vi "UHR-Fleezers Control (host) - 12.4.vi"() -> ()   [LabVIEW 2012] (continued)
            n735 = property on="Trap 1 (ON/OFF)" class="Bool (strict)"("Val(Sgnl)"=w1046) -> ()  [unwired: 2 in, 2 out]
            n736 = Array To Cluster(array=w1053) -> (cluster=w1052:cluster{"[0]":dbl, "[1]":dbl, "[2]":dbl})
            n737 = call "Set Stage Position.vi"("Position"=w1052, "error in"=w1047, "VISA resource name in"=w1048) -> ("error out"=w1051:errorcluster)  [unwired: 2 out]
            n738 = local write "Stage Control Serial Error"(w1051) -> ()
          }
          frame #2 {
            n739 = local write "Stage Moving"(FALSE ("Stage Moving")) -> ()
            n740 = call <vilib>:"Beep.vi"() -> ()  [unwired: 3 in, 9 out]
            n741 = case shown="True" "Cap 2 Flow ON" {
              frame False {
              }
              frame True {
                n742 = property on="Inject Pump 3" class="Bool (strict)"("Val(Sgnl)"=TRUE ("Value (Signaling)")) -> ()  [unwired: 2 in, 2 out]
              }
            }
          }
          frame #3 {
            n743 = property on="Sample Channel\nFlow" class="Bool (strict)"("Val(Sgnl)"=FALSE ("Value (Signaling)")) -> ()  [unwired: 2 in, 2 out]
            n744 = case shown="False" "Cap. 2 BD T1?\n(ADig T1, DNA T2)" {
              tunnel: "Cap 2 T ON" -> [w1067 w1068]
              frame False {
                n745 = property on="Trap 2 (ON/OFF)" class="Bool (strict)"("Val(Sgnl)"=w1067) -> ()  [unwired: 2 in, 2 out]
              }
              frame True {
                n746 = property on="Trap 1 (ON/OFF)" class="Bool (strict)"("Val(Sgnl)"=w1068) -> ()  [unwired: 2 in, 2 out]
              }
            }
            n747 = property on="Got ADig bead" class="Bool"("Key Focus"=TRUE) -> ()  [unwired: 2 in, 2 out]
          }
        }
      }
      event "Initialize Blue Laser": Value Change {
        n748 = event-data() -> ()  [unwired: 1 in, 5 out]
        n749 = flat-sequence {
          tunnel: w1069 -> [w1088]
          frame #0 {
            n750 = Concatenate Strings("slmp ", "Modulation\nPower (mW)") -> (w1087:string)
            n751 = call "serial write macro.vi"("String"=w1087, "Delay (ms)"="Delay (ms)", "VISA resource name"=w1088) -> ("read buffer"=w1076:string, "error out"=w1077:errorcluster, "VISA resource name out"=w1084:refnum<visa-resource-name>)
            n752 = local write "read blue buffer"(w1076) -> ()
            n753 = local write "Blue Error Out"(w1077) -> ()
            n754 = call "serial write macro.vi"("String"="sdmes 1", "Delay (ms)"="Delay (ms)", "VISA resource name"=w1084) -> ("read buffer"=w1074:string, "error out"=w1075:errorcluster, "VISA resource name out"=w1082:refnum<visa-resource-name>)
            n755 = local write "Blue Error Out"(w1075) -> ()
            n756 = local write "read blue buffer"(w1074) -> ()
            n757 = call "serial write macro.vi"("String"="sames 1", "Delay (ms)"="Delay (ms)", "VISA resource name"=w1082) -> ("read buffer"=w1071:string, "error out"=w1073:errorcluster, "VISA resource name out"=w1079:refnum<visa-resource-name>)
            n758 = local write "read blue buffer"(w1071) -> ()
            n759 = local write "Blue Error Out"(w1073) -> ()
            n760 = call "serial write macro.vi"("String"="l1", "Delay (ms)"="Delay (ms)", "VISA resource name"=w1079) -> ("read buffer"=w1070:string, "error out"=w1072:errorcluster)  [unwired: 1 out]
            n761 = local write "read blue buffer"(w1070) -> ()
            n762 = local write "Blue Error Out"(w1072) -> ()
          }
          frame #1 {
            n763 = local write "Initialize Blue Laser"(FALSE ("Initialize")) -> ()
          }
        }
      }
      event "Send string\nto Blue Laser": Value Change {
        n764 = event-data() -> ()  [unwired: 1 in, 5 out]
        n765 = flat-sequence {
          tunnel: w1090 -> [w1095]
          frame #0 {
            n766 = local read "Delay (ms)"() -> (w1092:i32)
            n767 = call "serial write macro.vi"("String"="command string", "Delay (ms)"=w1092, "VISA resource name"=w1095) -> ("read buffer"=w1093:string, "error out"=→"Blue Error Out":errorcluster)  [unwired: 1 out]
            "read blue buffer" <- w1093
            n768 = String Length(string=w1093) -> (length=→"length":i32)
            "command string sent" <- "command string"
          }
          frame #1 {
            n769 = local write "Send string\nto Blue Laser"(FALSE ("Send string")) -> ()
          }
        }
      }
      event "Read Harvard": Value Change {
        n770 = event-data() -> ()  [unwired: 1 in, 5 out]
        n771 = Concatenate Strings("write buffer", "\r") -> (w1102:string)
        n772 = VISA Write(VISA resource name=w1100, write buffer=w1102, error in (no error)=w1099) -> (VISA resource name out=w1111:refnum<visa-resource-name>, error out=w1110:errorcluster)  [unwired: 1 out]
        n773 = stacked-sequence {
          tunnel: [w1114] -> w1109
          tunnel: w1111 -> [w1114]
          tunnel: w1110 -> [w1113]
          tunnel: [w1113] -> w1104
          frame #0 {
            n774 = Wait (ms)(milliseconds to wait=50) -> ()  [unwired: 1 out]
          }
        }
        n775 = property class="Instr"(reference=w1109, error in=w1104) -> (reference out=w1108:refnum<visa-resource-name>, error out=w1106:errorcluster, "Serial Settings:Number of Bytes at Serial Port"=w1107:u32)
        "Serial Settings:Number of Bytes at Serial Port" <- w1107
        n776 = VISA Read(VISA resource name=w1108, byte count=w1107, error in (no error)=w1106) -> (read buffer=w1105:string)  [unwired: 3 out]
        "read buffer" <- w1105
        n777 = Fract/Exp String To Number(string=w1105) -> ()  [unwired: 5 out]
      }
      event "+z", "-z": Value Change {
        n778 = event-data() -> ()  [unwired: 1 in, 5 out]
        n779 = flat-sequence {
          tunnel: w1115 -> [w1137]
          tunnel: w1116 -> [w1117]
          frame #0 {
            n780 = call "Read Stage Position.vi"("error in"=w1137, "VISA resource name in"=w1117) -> ("Current Position"=w1122:cluster{dbl, dbl, dbl}, "error out"=w1135:errorcluster, "VISA resource name out"=w1136:refnum<visa-resource-name>)  [unwired: 1 out]
            n781 = local read "Saved Stage Positions"() -> (w1146:dbl[][])
            n782 = Divide(x="z nudge increment (um)", y=1000.0) -> (x/y=w1134:dbl)
            n783 = Boolean To (0,1)(Boolean="+z") -> (0, 1=w1126:i16)
            n784 = Boolean To (0,1)(Boolean="-z") -> (0, 1=w1127:i16)
            n785 = Array Subset(array=w1146, index (row)=1 ("index"), length (row)=1 ("length"), index (col)=1 ("index"), length (col)=3 ("length")) -> (w1143:dbl[][])
            n786 = Multiply(x=w1126, y=w1134) -> (x*y=w1130:dbl)
            n787 = Multiply(x=w1127, y=w1134) -> (x*y=w1128:dbl)
            n788 = Unbundle(w1122) -> (w1120:dbl, w1119:dbl, w1123:dbl)
            n789 = Negate(x=w1128) -> (-x=w1129:dbl)
            n790 = Reshape Array(w1143, 3 ("dimension size")) -> (w1141:dbl[])
            n791 = Add(x=w1130, y=w1129) -> (x+y=w1131:dbl)
            n792 = Array To Cluster(array=w1141) -> ()  [unwired: 1 out]
            n793 = Add(x=w1131, y=w1123) -> (x+y=w1121:dbl)
            n794 = Bundle(cluster=w1122, w1120, w1119, w1121) -> (w1118:cluster{dbl, dbl, dbl})
            n795 = call "Set Stage Position.vi"("Position"=w1118, "error in"=w1135, "VISA resource name in"=w1136) -> ("error out"=w1140:errorcluster)  [unwired: 2 out]
            n796 = local write "Stage Moving"(TRUE ("Stage Moving")) -> ()
            n797 = local write "Stage Control Serial Error"(w1140) -> ()
          }
          frame #1 {
            n798 = local write "Stage Moving"(FALSE ("Stage Moving")) -> ()
            n799 = call <vilib>:"Beep.vi"() -> ()  [unwired: 3 in, 9 out]
          }
        }
      }
      event "Cal/Data Acq. Spot": Value Change {
        n800 = event-data() -> ()  [unwired: 1 in, 5 out]
        n801 = flat-sequence {
          tunnel: w1155 -> [w1159]
          tunnel: w1156 -> [w1160]
          tunnel: [w1160] -> w1152
          tunnel: [w1159] -> w1151
          tunnel: w1152 -> [w1165]
          tunnel: w1151 -> [w1164]
          tunnel: ["Cal @ (MHz)"] -> w1149
          tunnel: [w1169] -> w1153
          tunnel: w1149 -> [w1169]
          tunnel: w1153 -> [w1178]
          tunnel: ["W/ Offset 1"] -> w1150
          tunnel: w1153 -> [w1199]
          tunnel: w1150 -> [w1197]
          frame #0 {
            n802 = property on="Sample Channel\nFlow" class="Bool (strict)"("Val(Sgnl)"="Daq spot flow on") -> ()  [unwired: 2 in, 2 out]
            n803 = Wait (ms)(milliseconds to wait=u32 250) -> ()  [unwired: 1 out]
          }
          frame #1 {
            n804 = local read "Saved Stage Positions"() -> (w1162:dbl[][])
            n805 = property on="Trap Delta (MHz)" class="DigNum (strict)"("Val(Sgnl)"="Cal @ (MHz)") -> ()  [unwired: 2 in, 2 out]
            n806 = local write "Stage Moving"(TRUE ("Stage Moving")) -> ()
            n807 = call "move to saved stage position.vi"("error in"=w1164, "Stage VISA resource name in"=w1165, "Position"="Cal Stage Position", "Saved Stage Positions"=w1162) -> ("error out"=w1163:errorcluster)  [unwired: 1 out]
            n808 = local write "Stage Control Serial Error"(w1163) -> ()
          }
          frame #2 {
            n809 = local write "Stage Moving"(FALSE ("Stage Moving")) -> ()
            n810 = property on="Sample Channel\nFlow" class="Bool (strict)"("Val(Sgnl)"="Flow ON during cal?") -> ()  [unwired: 2 in, 2 out]
            n811 = call <vilib>:"Beep.vi"() -> ()  [unwired: 3 in, 9 out]
          }
          frame #3 {
            n812 = Wait (ms)(milliseconds to wait=u32 1000) -> ()  [unwired: 1 out]
          }
          frame #4 {
            n813 = property on="Save Calibration" class="Bool (strict)"("Val(Sgnl)"=TRUE ("Value (Signaling)")) -> ()  [unwired: 2 in, 2 out]
          }
          frame #5 {
            n814 = Wait (ms)(milliseconds to wait=u32 2000) -> ()  [unwired: 1 out]
          }
          frame #6 {
            # "Check to see if \nsaving done"
            n815 = while {
              stop <- w1174 stop-if-true
              n816 = local read "Saving..."() -> (w1175:bool)
              n817 = Wait (ms)(milliseconds to wait=u32 100) -> ()  [unwired: 1 out]
              n818 = Not(x=w1175) -> (.not. x?=w1174:bool)
            }
          }
          frame #7 {
            n819 = case shown="True" "W/ Offset 1" {
              tunnel: w1178 -> [_ w1179]
              frame False {
              }
              frame True {
                n820 = stacked-sequence {
                  tunnel: w1179 -> [_ _ _ _ _ _ _ w1196]
                  frame #0 {
                    n821 = property on="Trap Delta (MHz)" class="DigNum (strict)"("Val(Sgnl)"="Offset 1 Start (MHz)") -> ()  [unwired: 2 in, 2 out]
                    n822 = Replace Array Subset(array=u32[] [0] ("Index Values"), new element="Offset 1 Set", index=0) -> (w1180:u32[])
                    n823 = property on="Saved AOD Raster Scan Parameter Sets" class="Arr (strict)"("Index Values"=w1180) -> ()  [unwired: 2 in, 2 out]
                  }
                  frame #1 {
                    n824 = Wait (ms)(milliseconds to wait=u32 200) -> ()  [unwired: 1 out]
                  }
                  frame #2 {
                    n825 = property on="Load parameters" class="Bool (strict)"("Val(Sgnl)"=TRUE ("Value (Signaling)")) -> ()  [unwired: 2 in, 2 out]
                  }
                  frame #3 {
                    n826 = Wait (ms)(milliseconds to wait=u32 200) -> ()  [unwired: 1 out]
                  }
                  frame #4 {
                    n827 = property on="Trap Raster Scan" class="Bool (strict)"("Val(Sgnl)"=TRUE ("Value (Signaling)")) -> ()  [unwired: 2 in, 2 out]
                  }
                  frame #5 {
                    n828 = Wait (ms)(milliseconds to wait=u32 2000) -> ()  [unwired: 1 out]
                  }
                  frame #6 {
                    n829 = while {
                      stop <- w1193 stop-if-true
                      n830 = local read "Raster Scanning..."() -> (w1195:bool)
                      n831 = local read "Saving..."() -> (w1191:bool)
                      n832 = Wait (ms)(milliseconds to wait=u32 100) -> ()  [unwired: 1 out]
                      n833 = Not(x=w1191) -> (.not. x?=w1190:bool)
                      n834 = Not(x=w1195) -> (.not. x?=w1192:bool)
                      n835 = And(x=w1192, y=w1190) -> (x .and. y?=w1193:bool)
                    }
                  }
                  frame #7 {
                    n836 = property on="Trap Delta (MHz)" class="DigNum (strict)"("Val(Sgnl)"=w1196) -> ()  [unwired: 2 in, 2 out]
                  }
                }
              }
            }
          }
          frame #8 {
            n837 = local read "Save ave N"() -> (w1198:dbl)
            n838 = case shown="False" "W/ Offset 2" {
              tunnel: w1199 -> [_ w1206]
              tunnel: w1198 -> [_ w1205]
              tunnel: w1197 -> [w1201 _]
              frame False {
                n839 = case shown="False" w1201 {
                  frame False {
                    n840 = Multiply(x="Cal read wait (s)", y=u32 1000 ("milliseconds to wait")) -> (x*y=w1203:u32)
                    n841 = Wait (ms)(milliseconds to wait=w1203) -> ()  [unwired: 1 out]
                  }
                  frame True {
                  }
                }
              }
              frame True {
                n842 = stacked-sequence {
                  tunnel: w1206 -> [_ _ _ _ _ _ _ _ _ w1227 _ _]
                  tunnel: w1205 -> [_ _ _ _ _ _ _ _ _ w1225 _ _]
                  frame #0 {
                    n843 = property on="Save ave N" class="DigNum (strict)"("Val(Sgnl)"=1.0 ("Value (Signaling)")) -> ()  [unwired: 2 in, 2 out]
                  }
                  frame #1 {
                    n844 = Wait (ms)(milliseconds to wait=u32 500) -> ()  [unwired: 1 out]
                  }
                  frame #2 {
                    n845 = property on="Trap Delta (MHz)" class="DigNum (strict)"("Val(Sgnl)"="Offset 2 Start (MHz)") -> ()  [unwired: 2 in, 2 out]
                    n846 = Replace Array Subset(array=u32[] [0] ("Index Values"), new element="Offset 2 Set", index=0) -> (w1211:u32[])
                    n847 = property on="Saved AOD Raster Scan Parameter Sets" class="Arr (strict)"("Index Values"=w1211) -> ()  [unwired: 2 in, 2 out]
                  }
                  frame #3 {
                    n848 = Wait (ms)(milliseconds to wait=u32 500) -> ()  [unwired: 1 out]
                  }
                  frame #4 {
                    n849 = property on="Load parameters" class="Bool (strict)"("Val(Sgnl)"=TRUE ("Value (Signaling)")) -> ()  [unwired: 2 in, 2 out]
                  }
                  frame #5 {
                    n850 = Wait (ms)(milliseconds to wait=u32 500) -> ()  [unwired: 1 out]
                  }
                  frame #6 {
                    n851 = property on="Trap Raster Scan" class="Bool (strict)"("Val(Sgnl)"=TRUE ("Value (Signaling)")) -> ()  [unwired: 2 in, 2 out]
                  }
                  frame #7 {
                    n852 = Wait (ms)(milliseconds to wait=u32 2000) -> ()  [unwired: 1 out]
                  }
                  frame #8 {
                    n853 = while {
                      stop <- w1220 stop-if-true
                      n854 = local read "Raster Scanning..."() -> (w1223:bool)
                      n855 = local read "Saving..."() -> (w1221:bool)
                      n856 = Wait (ms)(milliseconds to wait=u32 100) -> ()  [unwired: 1 out]
                      n857 = Not(x=w1221) -> (.not. x?=w1219:bool)
                      n858 = Not(x=w1223) -> (.not. x?=w1222:bool)
                      n859 = And(x=w1222, y=w1219) -> (x .and. y?=w1220:bool)
                    }
                  }
                  frame #9 {
                    n860 = property on="Trap Delta (MHz)" class="DigNum (strict)"("Val(Sgnl)"=w1227) -> ()  [unwired: 2 in, 2 out]
                    n861 = property on="Saved AOD Raster Scan Parameter Sets" class="Arr (strict)"("Index Values"=u32[] [0]) -> ()  [unwired: 2 in, 2 out]
                    n862 = property on="Save ave N" class="DigNum (strict)"("Val(Sgnl)"=w1225) -> ()  [unwired: 2 in, 2 out]
                  }
                  frame #10 {
                    n863 = Wait (ms)(milliseconds to wait=u32 500) -> ()  [unwired: 1 out]
                  }
                  frame #11 {
                    n864 = property on="Load parameters" class="Bool (strict)"("Val(Sgnl)"=TRUE ("Value (Signaling)")) -> ()  [unwired: 2 in, 2 out]
                  }
                }
              }
            }
          }
          frame #9 {
            n865 = property on="Read Cal" class="Bool (strict)"("Val(Sgnl)"=TRUE ("Value (Signaling)")) -> ()  [unwired: 2 in, 2 out]
          }
          frame #10 {
            n866 = Wait (ms)(milliseconds to wait=u32 1000) -> ()  [unwired: 1 out]
          }
          frame #11 {
            n867 = property on="Fish for Tether" class="Bool (strict)"("Val(Sgnl)"=TRUE ("Value (Signaling)")) -> ()  [unwired: 2 in, 2 out]
          }
        }
        n868 = local write "Cal/Data Acq. Spot"(FALSE ("Cal/Data Acq. Spot")) -> ()
      }
      event "Dump Beads": Value Change {
        n869 = event-data() -> ()  [unwired: 1 in, 5 out]
        n870 = flat-sequence {
          tunnel: ["Dump spot flow on?"] -> w1233
          tunnel: [w1244] -> w1234
          tunnel: w1233 -> [w1244]
          tunnel: w1237 -> [w1249]
          tunnel: w1236 -> [w1248]
          tunnel: [w1246] -> w1235
          tunnel: w1234 -> [w1246]
          tunnel: w1235 -> [w1259]
          frame #0 {
            w1238 = FALSE ("Value (Signaling)")
            n871 = local read "Saving..."() -> (w1240:bool)
            n872 = local write "Dump Beads"(FALSE ("Dump Beads")) -> ()
            n873 = property on="Inject Pump 3" class="Bool (strict)"("Val(Sgnl)"=w1238) -> ()  [unwired: 2 in, 2 out]
            n874 = property on="Inject Pump 1" class="Bool (strict)"("Val(Sgnl)"=w1238) -> ()  [unwired: 2 in, 2 out]
            n875 = local write "Stop Saving"(w1240) -> ()
          }
          frame #1 {
            w1241 = FALSE ("Fl. Triggered...")
            n876 = case shown="True" "Dump spot flow on?" {
              frame False {
              }
              frame True {
                n877 = property on="Sample Channel\nFlow" class="Bool (strict)"("Val(Sgnl)"=TRUE ("Stage Moving")) -> ()  [unwired: 2 in, 2 out]
              }
            }
            n878 = local write "Fl. Triggered..."(w1241) -> ()
            n879 = local write "Tether"(w1241) -> ()
            n880 = property on="Green Laser ON" class="Bool (strict)"("Val(Sgnl)"=w1241) -> ()  [unwired: 2 in, 2 out]
            n881 = property on="Trap Pos. FB ON" class="Bool (strict)"("Val(Sgnl)"=w1241) -> ()  [unwired: 2 in, 2 out]
            n882 = property on="Trap Trig. Fl." class="Bool (strict)"("Val(Sgnl)"=w1241) -> ()  [unwired: 2 in, 2 out]
            n883 = property on="Fl. Triggered..." class="Bool (strict)"("Val(Sgnl)"=w1241) -> ()  [unwired: 2 in, 2 out]
            n884 = property on="Dip for Protein" class="Bool (strict)"("Val(Sgnl)"=w1241) -> ()  [unwired: 2 in, 2 out]
            n885 = property on="Pause dwell" class="Bool (strict)"("Val(Sgnl)"=w1241) -> ()  [unwired: 2 in, 2 out]
          }
          frame #2 {
            n886 = property on="Trap Pos. FB Offset Factor" class="DigNum (strict)"("Val(Sgnl)"=i64 0 ("Value (Signaling)")) -> ()  [unwired: 2 in, 2 out]
          }
          frame #3 {
            n887 = local read "Saved Stage Positions"() -> (w1250:dbl[][])
            n888 = local write "Stage Moving"(TRUE ("Stage Moving")) -> ()
            n889 = Array Subset(array=w1250, index (row)=3 ("index"), length (row)=1 ("length"), index (col)=1 ("index"), length (col)=3 ("length")) -> (w1255:dbl[][])
            n890 = Reshape Array(w1255, 3 ("dimension size")) -> (w1253:dbl[])
            n891 = Array To Cluster(array=w1253) -> (cluster=w1252:cluster{"[0]":dbl, "[1]":dbl, "[2]":dbl})
            n892 = call "Set Stage Position.vi"("Position"=w1252, "error in"=w1248, "VISA resource name in"=w1249) -> ()  [unwired: 3 out]
          }
          frame #4 {
            w1260 = FALSE ("Value (Signaling)")
            n893 = case shown="True" w1259 {
              frame False {
              }
              frame True {
                n894 = property on="Sample Channel\nFlow" class="Bool (strict)"("Val(Sgnl)"=FALSE ("Stage Moving")) -> ()  [unwired: 2 in, 2 out]
              }
            }
            n895 = property on="Trap 1 (ON/OFF)" class="Bool (strict)"("Val(Sgnl)"=w1260) -> ()  [unwired: 2 in, 2 out]
            n896 = property on="Trap 2 (ON/OFF)" class="Bool (strict)"("Val(Sgnl)"=w1260) -> ()  [unwired: 2 in, 2 out]
            n897 = call <vilib>:"Beep.vi"() -> ()  [unwired: 3 in, 9 out]
          }
          frame #5 {
            n898 = property on="Move Cap. 2 (ADig Top)" class="Bool (strict)"("Val(Sgnl)"=TRUE ("Value (Signaling)")) -> ()  [unwired: 2 in, 2 out]
            n899 = property on="Tab Control" class="TabCtl (strict)"("Val(Sgnl)"=T25."Status" ("Value (Signaling)")) -> ()  [unwired: 2 in, 2 out]
          }
        }
      }
      event "Dip for Protein": Value Change {
        n900 = event-data() -> ()  [unwired: 1 in, 5 out]
        n901 = case shown="True" "Dip for Protein" {
          tunnel: w1266 -> [_ w1268]
          tunnel: w1265 -> [_ w1267]
          frame False {
          }
          frame True {
            n902 = while {
              tunnel: w1268 -> [w1279]
              tunnel: w1267 -> [w1278]
              i -> [w1273]
              stop <- w1275 stop-if-true
              n903 = Increment(x=w1273) -> (x+1=→"Dip #":i32)
              n904 = flat-sequence {
                tunnel: w1278 -> [w1290]
                tunnel: w1279 -> [w1291]
                tunnel: [w1291] -> w1283
                tunnel: [w1290] -> w1282
                tunnel: [w1284] -> w1269
                tunnel: [w1296] -> w1277
                tunnel: [w1297] -> w1276
                tunnel: w1283 -> [w1298]
                tunnel: w1282 -> [w1299]
                tunnel: [w1294] -> w1270
                tunnel: w1269 -> [w1294]
                tunnel: [w1307] -> w1281
                tunnel: w1277 -> [w1307]
                tunnel: [w1306] -> w1280
                tunnel: w1276 -> [w1306]
                tunnel: [w1303] -> w1274
                tunnel: [w1302] -> w1271
                tunnel: w1270 -> [w1302]
                tunnel: w1280 -> [w1327]
                tunnel: w1281 -> [w1328]
                tunnel: w1274 -> [w1329]
                tunnel: w1271 -> [w1326]
                tunnel: [w1385] -> w1275
                frame #0 {
                  n905 = local read "Trap Pos. FB ON"() -> (w1284:bool)
                  n906 = Compound Arithmetic op=AND("Flow ON\nduring dip?", "FB OFF when \nflow ON", w1284) -> (w1285:bool)
                  n907 = case shown="True" "Move trap \nbefore dip move?" {
                    frame False {
                    }
                    frame True {
                      n908 = property on="Trap Delta (MHz)" class="DigNum (strict)"("Val(Sgnl)"="Dipping Delta (MHz)") -> ()  [unwired: 2 in, 2 out]
                    }
                  }
                  n909 = property on="Green Laser ON" class="Bool (strict)"("Val(Sgnl)"="Green ON\nbefore dip?") -> ()  [unwired: 2 in, 2 out]
                  n910 = property on="Sample Channel\nFlow" class="Bool (strict)"("Val(Sgnl)"="Flow ON\nduring dip?") -> ()  [unwired: 2 in, 2 out]
                  n911 = case shown="True" w1285 {
                    frame False {
                    }
                    frame True {
                      n912 = property on="Trap Pos. FB ON" class="Bool (strict)"("Val(Sgnl)"=FALSE ("Value (Signaling)")) -> ()  [unwired: 2 in, 2 out]
                    }
                  }
                }
                frame #1 {
                  n913 = local read "Saved Stage Positions"() -> (w1301:dbl[][])
                  n914 = local write "Cancel dwell"(FALSE ("Cancel dwell")) -> ()
                  n915 = call "move to saved stage position.vi"("error in"=w1299, "Stage VISA resource name in"=w1298, "Position"="Dip Stage \nPosition", "Saved Stage Positions"=w1301) -> ("VISA resource name out"=w1296:refnum<visa-resource-name>, "error out"=w1297:errorcluster)
                }
                frame #2 {
                  n916 = node-c288() -> (w1305:T22)  [unwired: 4 in]
                  n917 = timed-loop {
                    timing: w1305 -> [_]
                    timing-out: [_] -> w1304
                    tunnel: [w1311] -> w1303
                    i -> [w1308]
                    stop <- w1312 stop-if-true
                    n918 = node-c288() -> ()  [unwired: 1 in, 1 out]
                    n919 = Greater Or Equal?(x=w1308, y="Dip Duration (s)") -> (x >= y?=w1320:bool)
                    n920 = local read "Dip for Protein"() -> (w1313:bool)
                    n921 = local read "Dump Beads"() -> (w1310:bool)
                    n922 = local read "Cancel dwell"() -> (w1319:bool)
                    n923 = local read "Pause dwell"() -> (w1316:bool)
                    n924 = Not(x=w1313) -> (.not. x?=w1318:bool)
                    n925 = Compound Arithmetic op=OR(w1319, w1320, w1318) -> (w1317:bool)
                    n926 = Select(t=FALSE, s=w1316, f=w1317) -> (s? t:f=w1314:bool)
                    n927 = Not(x=w1310) -> (.not. x?=w1309:bool)
                    n928 = node-c288() -> ()  [unwired: 1 in, 1 out]
                    n929 = And(x=w1313, y=w1309) -> (x .and. y?=w1311:bool)
                    n930 = Or(x=w1314, y=w1310) -> (x .or. y?=w1312:bool)
                    "Dip Time (s)" <- w1308
                  }
                  n931 = node-c288(w1304) -> ()  [unwired: 1 out]
                }
                frame #3 {
                  n932 = case shown="True" w1329 {
                    tunnel: w1328 -> [_ w1334]
                    tunnel: w1327 -> [_ w1333]
                    tunnel: w1326 -> [_ w1330]
                    frame False {
                    }
                    frame True {
                      n933 = flat-sequence {
                        tunnel: w1333 -> [w1338]
                        tunnel: w1334 -> [w1339]
                        tunnel: [w1339] -> w1332
                        tunnel: [w1338] -> w1331
                        tunnel: w1330 -> [w1335]
                        tunnel: w1332 -> [w1349]
                        tunnel: w1331 -> [w1348]
                        tunnel: w1330 -> [w1357]
                        frame #0 {
                          n934 = local read "Sample Channel\nFlow"() -> (w1337:bool)
                          n935 = case shown="True" w1337 {
                            tunnel: "Flow ON \nduring return\nfrom dip?" -> [w1340 w1343]
                            tunnel: w1335 -> [_ w1342]
                            frame False {
                              n936 = case shown="True" w1340 {
                                frame False {
                                }
                                frame True {
                                n937 = property on="Sample Channel\nFlow" class="Bool (strict)"("Val(Sgnl)"=TRUE ("Value (Signaling)")) -> ()  [unwired: 2 in, 2 out]
                                }
                              }
                            }
                            frame True {
                              n938 = case shown="False" w1343 {
                                tunnel: w1342 -> [w1344 _]
                                frame False {
                                n939 = property on="Trap Pos. FB ON" class="Bool (strict)"("Val(Sgnl)"=w1344) -> ()  [unwired: 2 in, 2 out]
                                n940 = property on="Sample Channel\nFlow" class="Bool (strict)"("Val(Sgnl)"=FALSE ("Value (Signaling)")) -> ()  [unwired: 2 in, 2 out]
                                }
                                frame True {
                                }
                              }
                            }
                          }
                        }
                        frame #1 {
                          # "For turning on green laser before stage reaches lower spot"
                          n941 = case shown="True" "Green ON\nafter start\nreturn?" {
                            frame False {
                            }
                            frame True {
                              n942 = flat-sequence {
                                frame #0 {
                                n943 = Multiply(x="Green delay after \nstart return (s)", y=1000.0) -> (x*y=w1354:dbl)
                                n944 = Wait (ms)(milliseconds to wait=w1354) -> ()  [unwired: 1 out]
                                }
                                frame #1 {
                                n945 = property on="Green Laser ON" class="Bool (strict)"("Val(Sgnl)"=TRUE ("Value (Signaling)")) -> ()  [unwired: 2 in, 2 out]
                                }
                              }
                            }
                          }
                          n946 = local read "Saved Stage Positions"() -> (w1352:dbl[][])
                          n947 = local write "Cancel dwell"(FALSE ("Cancel dwell")) -> ()
                          n948 = call "move to saved stage position.vi"("error in"=w1348, "Stage VISA resource name in"=w1349, "Position"="Return Stage \nPosition", "Saved Stage Positions"=w1352) -> ("error out"=w1350:errorcluster)  [unwired: 1 out]
                          n949 = local write "Stage Control Serial Error"(w1350) -> ()
                        }
                        frame #2 {
                          n950 = property on="Trap Pos. FB ON" class="Bool (strict)"("Val(Sgnl)"=w1357) -> ()  [unwired: 2 in, 2 out]
                          n951 = case shown="True" "Green ON \nafter return?" {
                            frame False {
                            }
                            frame True {
                              n952 = property on="Green Laser ON" class="Bool (strict)"("Val(Sgnl)"=TRUE ("Value (Signaling)")) -> ()  [unwired: 2 in, 2 out]
                            }
                          }
                          n953 = case shown="True" "Move trap after return?" {
                            frame False {
                            }
                            frame True {
                              n954 = property on="Trap Delta (MHz)" class="DigNum (strict)"("Val(Sgnl)"="Dip Trap Delta 2 (MHz)") -> ()  [unwired: 2 in, 2 out]
                            }
                          }
                          n955 = case shown="True" "Save data after return?" {
                            frame False {
                            }
                            frame True {
                              n956 = property on="Start Saving" class="Bool (strict)"("Val(Sgnl)"=TRUE ("Value (Signaling)")) -> ()  [unwired: 2 in, 2 out]
                            }
                          }
                          n957 = property on="Sample Channel\nFlow" class="Bool (strict)"("Val(Sgnl)"="Flow ON\nduring daq?") -> ()  [unwired: 2 in, 2 out]
                        }
                        frame #3 {
                          n958 = node-c288() -> (w1366:T22)  [unwired: 4 in]
                          n959 = timed-loop {
                            timing: w1366 -> [_]
                            timing-out: [_] -> w1365
                            i -> [w1367]
                            stop <- w1369 stop-if-true
                            n960 = node-c288() -> ()  [unwired: 1 in, 1 out]
                            n961 = local read "Dump Beads"() -> (w1368:bool)
                            n962 = Greater Or Equal?(x=w1367, y="Dwell Duration (s)") -> (x >= y?=w1374:bool)
                            n963 = local read "Dip for Protein"() -> (w1371:bool)
                            n964 = Not(x=w1371) -> (.not. x?=w1370:bool)
                            n965 = Compound Arithmetic op=OR(w1374, "Cancel dwell", w1370) -> (w1373:bool)
                            n966 = node-c288() -> ()  [unwired: 1 in, 1 out]
                            n967 = Select(t=FALSE, s="Pause dwell", f=w1373) -> (s? t:f=w1376:bool)
                            n968 = Or(x=w1376, y=w1368) -> (x .or. y?=w1369:bool)
                            "Dwell Time (s)" <- w1367
                          }
                          n969 = node-c288(w1365) -> ()  [unwired: 1 out]
                        }
                      }
                    }
                  }
                }
                frame #4 {
                  n970 = local read "Dip for Protein"() -> (w1386:bool)
                  n971 = local read "Dump Beads"() -> (w1383:bool)
                  n972 = local write "Cancel dwell"(FALSE ("Cancel dwell")) -> ()
                  n973 = Not(x=w1386) -> (.not. x?=w1387:bool)
                  n974 = Not(x="Cont. Repeat Dipping?") -> (.not. x?=w1389:bool)
                  n975 = Compound Arithmetic op=OR(w1387, w1389, w1383) -> (w1385:bool)
                }
              }
            }
          }
        }
      }
      event "Profile": Value Change {
        n976 = event-data() -> ()  [unwired: 1 in, 5 out]
        n977 = flat-sequence {
          tunnel: w1398 -> [w1401]
          tunnel: w1397 -> [w1409]
          tunnel: [w1403] -> w1396
          tunnel: [w1402] -> w1395
          tunnel: [w1400] -> w1393
          tunnel: [w1399] -> w1390
          tunnel: w1396 -> [w1416]
          tunnel: w1395 -> [w1415]
          tunnel: [w1413] -> w1394
          tunnel: w1393 -> [w1414]
          tunnel: [w1412] -> w1392
          tunnel: [w1411] -> w1391
          tunnel: w1390 -> [w1411]
          tunnel: w1394 -> [w1420]
          tunnel: w1392 -> [w1419]
          tunnel: w1391 -> [w1418]
          frame #0 {
            n978 = call "Read Stage Position.vi"("error in"=w1409, "VISA resource name in"=w1401) -> ("Current Position"=w1399:cluster{dbl, dbl, dbl}, "error out"=w1402:errorcluster, "VISA resource name out"=w1400:refnum<visa-resource-name>)  [unwired: 1 out]
            "Current Position" <- w1399
            n979 = local write "Stage Control Serial Error"(w1402) -> ()
            n980 = Unbundle(w1399) -> (w1406:dbl, w1408:dbl, w1404:dbl)
            n981 = Add(x=w1408, y="Y change (mm)") -> (x+y=w1405:dbl)
            n982 = Bundle(w1406, w1405, w1404) -> (w1403:cluster{dbl, dbl, dbl})  [unwired: 1 in]
          }
          frame #1 {
            # "move to new position and start saving"
            n983 = local write "Stage Moving"(TRUE ("Stage Moving")) -> ()
            n984 = local write "Start Saving"(TRUE ("Start Saving")) -> ()
            n985 = call "Set Stage Position.vi"("Position"=w1416, "error in"=w1415, "VISA resource name in"=w1414) -> ("error out"=w1412:errorcluster, "VISA resource name out"=w1413:refnum<visa-resource-name>)  [unwired: 1 out]
          }
          frame #2 {
            # "go back to start"
            n986 = call "Set Stage Position.vi"("Position"=w1418, "error in"=w1419, "VISA resource name in"=w1420) -> ()  [unwired: 3 out]
          }
          frame #3 {
            # "stop saving"
            n987 = local write "Stop Saving"(TRUE ("Stop Saving")) -> ()
            n988 = local write "Stage Moving"(FALSE ("Stage Moving")) -> ()
          }
        }
      }
      event "Move to Position 1", "Move to Position 2", "Move to Position 3", "Move to Position 4", "Move to Position 5", "Lower Ch. Cap.": Value Change {
        n989 = event-data() -> ()  [unwired: 1 in, 5 out]
        n990 = Or(x="Move to Position 5", y="Lower Ch. Cap.") -> (x .or. y?=w1426:bool)
        n991 = Build Array("Move to Position 1", "Move to Position 2", "Move to Position 3", "Move to Position 4", w1426) -> (w1429:bool[])
        n992 = Boolean Array To Number(Boolean array=w1429) -> (number=w1428:u32)
        n993 = Logarithm Base 2(1:w1428) -> (0:w1427:dbl)
        n994 = flat-sequence {
          tunnel: w1427 -> [w1438]
          tunnel: w1424 -> [w1436]
          tunnel: w1423 -> [w1435]
          frame #0 {
            n995 = local read "Saved Stage Positions"() -> (w1446:dbl[][])
            n996 = Array Subset(array=w1446, index (row)=w1438, length (row)=1 ("length"), index (col)=1 ("index"), length (col)=3 ("length")) -> (w1443:dbl[][])
            n997 = Reshape Array(w1443, 3 ("dimension size")) -> (w1441:dbl[])
            n998 = Array To Cluster(array=w1441) -> (cluster=w1440:cluster{"[0]":dbl, "[1]":dbl, "[2]":dbl})
            n999 = call "Set Stage Position.vi"("Position"=w1440, "error in"=w1435, "VISA resource name in"=w1436) -> ("error out"=w1439:errorcluster)  [unwired: 2 out]
            n1000 = local write "Stage Moving"(TRUE ("Stage Moving")) -> ()
            n1001 = local write "Stage Control Serial Error"(w1439) -> ()
          }
          frame #1 {
            n1002 = local write "Stage Moving"(FALSE ("Stage Moving")) -> ()
            n1003 = call <vilib>:"Beep.vi"() -> ()  [unwired: 3 in, 9 out]
          }
        }
      }
      event "Got ADig bead": Value Change {
        n1004 = event-data() -> ()  [unwired: 1 in, 5 out]
        n1005 = flat-sequence {
          frame #0 {
            n1006 = local read "Cap 1 Samp Flow ON"() -> (w1450:bool)
            n1007 = case shown="True" w1450 {
              frame False {
              }
              frame True {
                n1008 = property on="Sample Channel\nFlow" class="Bool (strict)"("Val(Sgnl)"=TRUE ("Value (Signaling)")) -> ()  [unwired: 2 in, 2 out]
              }
            }
          }
          frame #1 {
            n1009 = property on="Inject Pump 3" class="Bool (strict)"("Val(Sgnl)"=FALSE ("Value (Signaling)")) -> ()  [unwired: 2 in, 2 out]
          }
          frame #2 {
            n1010 = property on="Move Cap. 1 (DNA Bottom)" class="Bool (strict)"("Val(Sgnl)"=TRUE ("Value (Signaling)")) -> ()  [unwired: 2 in, 2 out]
          }
        }
      }
      event "Force FB Data\nScript": Value Change {
        n1011 = event-data() -> ()  [unwired: 1 in, 5 out]
        n1012 = flat-sequence {
          tunnel: w1459 -> [w1463]
          tunnel: w1460 -> [w1464]
          tunnel: [w1464] -> w1455
          tunnel: [w1463] -> w1454
          tunnel: w1455 -> [w1467]
          tunnel: w1454 -> [w1466]
          tunnel: ["Trap Trig Fl."] -> w1456
          tunnel: [w1492] -> w1457
          tunnel: w1456 -> [w1492]
          tunnel: [w1496] -> w1458
          tunnel: w1457 -> [w1496]
          tunnel: w1458 -> [w1498]
          frame #0 {
            n1013 = property on="Trap Delta (MHz)" class="DigNum (strict)"("Val(Sgnl)"="Trap Delta Before Moving") -> ()  [unwired: 2 in, 2 out]
          }
          frame #1 {
            n1014 = local read "Saved Stage Positions"() -> (w1469:dbl[][])
            n1015 = local write "FB Trap Pos Offset"(0.0 ("FB Trap Pos Offset")) -> ()
            n1016 = property on="Trap Pos. FB Offset Factor" class="DigNum (strict)"("Val(Sgnl)"=i64 0 ("Value (Signaling)")) -> ()  [unwired: 2 in, 2 out]
            n1017 = local write "Stage Moving"(TRUE ("Stage Moving")) -> ()
            n1018 = call "move to saved stage position.vi"("error in"=w1466, "Stage VISA resource name in"=w1467, "Position"="Stage Position To Establish FB", "Saved Stage Positions"=w1469) -> ("error out"=w1465:errorcluster)  [unwired: 1 out]
            n1019 = local write "Stage Control Serial Error"(w1465) -> ()
          }
          frame #2 {
            n1020 = call <vilib>:"Beep.vi"() -> ()  [unwired: 3 in, 9 out]
            n1021 = Multiply(x="Wait (s)", y=u32 1000 ("milliseconds to wait")) -> (x*y=w1476:u32)
            n1022 = property on="Trap Delta (MHz)" class="DigNum (strict)"("Val(Sgnl)"="Starting \nTrap Delta (MHz)") -> ()  [unwired: 2 in, 2 out]
            n1023 = local write "Stage Moving"(FALSE ("Stage Moving")) -> ()
            n1024 = Wait (ms)(milliseconds to wait=w1476) -> ()  [unwired: 1 out]
            n1025 = property on="Tab Control 2" class="TabCtl (strict)"("Val(Sgnl)"=T6."Feedback on Trap Position" ("Value (Signaling)")) -> ()  [unwired: 2 in, 2 out]
            n1026 = property on="Tab Control" class="TabCtl (strict)"("Val(Sgnl)"=T4."Trap Control (RF)" ("Value (Signaling)")) -> ()  [unwired: 2 in, 2 out]
          }
          frame #3 {
            n1027 = property on="Set Reading to\nSetpoint" class="Bool (strict)"("Val(Sgnl)"=TRUE ("Value (Signaling)")) -> ()  [unwired: 2 in, 2 out]
            n1028 = Wait (ms)(milliseconds to wait=u32 500) -> ()  [unwired: 1 out]
          }
          frame #4 {
            n1029 = property on="Trap Pos. FB ON" class="Bool (strict)"("Val(Sgnl)"=TRUE ("Value (Signaling)")) -> ()  [unwired: 2 in, 2 out]
            n1030 = Wait (ms)(milliseconds to wait=u32 250) -> ()  [unwired: 1 out]
          }
          frame #5 {
            n1031 = case shown="False" "Trap Trig Fl." {
              frame False {
                n1032 = case shown="True" "Green ON after FB ON?" {
                  selector: "Green ON after FB ON?" -> [_ w1491]
                  frame False {
                  }
                  frame True {
                    n1033 = property on="Green Laser ON" class="Bool (strict)"("Val(Sgnl)"=w1491) -> ()  [unwired: 2 in, 2 out]
                  }
                }
              }
              frame True {
              }
            }
            n1034 = case shown="True" "Remove Action Offset" {
              tunnel: TRUE ("Value (Signaling)") -> [w1488 w1489]
              frame False {
                n1035 = property on="Remove Unwinding Offset" class="Bool (strict)"("Val(Sgnl)"=w1488) -> ()  [unwired: 2 in, 2 out]
              }
              frame True {
                n1036 = property on="Remove Action Offset" class="Bool (strict)"("Val(Sgnl)"=w1489) -> ()  [unwired: 2 in, 2 out]
              }
            }
            n1037 = Wait (ms)(milliseconds to wait=u32 250) -> ()  [unwired: 1 out]
          }
          frame #6 {
            n1038 = property on="Start Saving" class="Bool (strict)"("Val(Sgnl)"=TRUE ("Value (Signaling)")) -> ()  [unwired: 2 in, 2 out]
            n1039 = Wait (ms)(milliseconds to wait=u32 5000) -> ()  [unwired: 1 out]
          }
          frame #7 {
            w1495 = TRUE ("Value (Signaling)")
            n1040 = property on="Rem fb disp offset" class="Bool (strict)"("Val(Sgnl)"=w1495) -> ()  [unwired: 2 in, 2 out]
            n1041 = property on="Remove Offset" class="Bool (strict)"("Val(Sgnl)"=w1495) -> ()  [unwired: 2 in, 2 out]
            n1042 = Wait (ms)(milliseconds to wait=u32 100) -> ()  [unwired: 1 out]
          }
          frame #8 {
            n1043 = case shown="True" w1498 {
              frame False {
              }
              frame True {
                n1044 = local write "Trap Trig. Fl."(TRUE ("Value (Signaling)")) -> ()
              }
            }
          }
          frame #9 {
            n1045 = case shown="True" "Start dipping after?" {
              frame False {
              }
              frame True {
                n1046 = flat-sequence {
                  frame #0 {
                    n1047 = Multiply(x="Delay before dipping (s)", y=1000.0) -> (x*y=w1502:dbl)
                    n1048 = Wait (ms)(milliseconds to wait=w1502) -> ()  [unwired: 1 out]
                  }
                  frame #1 {
                    n1049 = property on="Dip for Protein" class="Bool (strict)"("Val(Sgnl)"=TRUE ("Value (Signaling)")) -> ()  [unwired: 2 in, 2 out]
                    n1050 = local write "Scripts"(T1."Dipping" ("Scripts")) -> ()
                  }
                }
              }
            }
          }
        }
      }
      event "Fixed Traps Data\nScript": Value Change {
        n1051 = event-data() -> ()  [unwired: 1 in, 5 out]
        n1052 = flat-sequence {
          frame #0 {
            n1053 = case shown="True" "Green ON" {
              frame False {
              }
              frame True {
                n1054 = property on="Green Laser ON" class="Bool (strict)"("Val(Sgnl)"=TRUE) -> ()  [unwired: 2 in, 2 out]
              }
            }
            n1055 = local write "Offset (nm)"(0.0 ("Offset (nm)")) -> ()
            n1056 = property on="Sample Channel\nFlow" class="Bool (strict)"("Val(Sgnl)"=FALSE ("Value (Signaling)")) -> ()  [unwired: 2 in, 2 out]
            n1057 = property on="Trap Delta (MHz)" class="DigNum (strict)"("Val(Sgnl)"="Fixed Traps Trap Delta (MHz)") -> ()  [unwired: 2 in, 2 out]
          }
          frame #1 {
            n1058 = Wait (ms)(milliseconds to wait=u32 1000) -> ()  [unwired: 1 out]
          }
          frame #2 {
            n1059 = local write "Start Saving"(TRUE ("Start Saving")) -> ()
          }
          frame #3 {
            n1060 = local read "Bead Sep. Int. Time (s)"() -> (w1513:dbl)
            n1061 = Multiply(x=w1513, y=1000.0) -> (x*y=w1515:dbl)
            n1062 = Wait (ms)(milliseconds to wait=w1515) -> ()  [unwired: 1 out]
          }
          frame #4 {
            n1063 = property on="Remove Offset" class="Bool (strict)"("Val(Sgnl)"=TRUE ("Value (Signaling)")) -> ()  [unwired: 2 in, 2 out]
          }
          frame #5 {
            n1064 = property on="Dip for Protein" class="Bool (strict)"("Val(Sgnl)"="Start dipping after?") -> ()  [unwired: 2 in, 2 out]
          }
        }
      }
      event "Got DNA bead": Value Change {
        n1065 = event-data() -> ()  [unwired: 1 in, 5 out]
        n1066 = flat-sequence {
          frame #0 {
            n1067 = local read "Daq spot flow on"() -> (w1520:bool)
            n1068 = case shown="True" w1520 {
              frame False {
              }
              frame True {
                n1069 = property on="Sample Channel\nFlow" class="Bool (strict)"("Val(Sgnl)"=TRUE ("Value (Signaling)")) -> ()  [unwired: 2 in, 2 out]
              }
            }
            n1070 = property on="Got DNA bead" class="Bool"("Key Focus"=FALSE) -> ()  [unwired: 2 in, 2 out]
          }
          frame #1 {
            n1071 = property on="Inject Pump 1" class="Bool (strict)"("Val(Sgnl)"=FALSE ("Value (Signaling)")) -> ()  [unwired: 2 in, 2 out]
          }
          frame #2 {
            n1072 = property on="Cal/Data Acq. Spot" class="Bool (strict)"("Val(Sgnl)"=TRUE ("Value (Signaling)")) -> ()  [unwired: 2 in, 2 out]
          }
        }
      }
      event "Take Stepping Data": Value Change {
        n1073 = event-data() -> ()  [unwired: 1 in, 5 out]
        n1074 = local read "Save ave N"() -> (w1532:dbl)
        n1075 = flat-sequence {
          tunnel: w1532 -> [w1534]
          tunnel: [w1534] -> w1527
          tunnel: [w1536] -> w1528
          tunnel: w1527 -> [w1536]
          tunnel: [w1538] -> w1529
          tunnel: w1528 -> [w1538]
          tunnel: [w1541] -> w1530
          tunnel: w1529 -> [w1541]
          tunnel: [w1543] -> w1531
          tunnel: w1530 -> [w1543]
          tunnel: [w1545] -> w1525
          tunnel: w1531 -> [w1545]
          tunnel: w1525 -> [w1548]
          tunnel: [w1548] -> w1524
          tunnel: w1524 -> [w1549]
          tunnel: [w1549] -> w1526
          tunnel: w1526 -> [w1555]
          frame #0 {
            n1076 = property on="Save ave N" class="DigNum (strict)"("Val(Sgnl)"="Save ave factor") -> ()  [unwired: 2 in, 2 out]
          }
          frame #1 {
            n1077 = Wait (ms)(milliseconds to wait=u32 100) -> ()  [unwired: 1 out]
          }
          frame #2 {
            n1078 = local read "Offset 2 Start (MHz)"() -> (w1540:dbl)
            n1079 = property on="Saved AOD Raster Scan Parameter Sets" class="Arr (strict)"("Index Values"=u32[] [2]) -> ()  [unwired: 2 in, 2 out]
            n1080 = property on="Trap Delta (MHz)" class="DigNum (strict)"("Val(Sgnl)"=w1540) -> ()  [unwired: 2 in, 2 out]
          }
          frame #3 {
            n1081 = property on="Load parameters" class="Bool (strict)"("Val(Sgnl)"=TRUE ("Value (Signaling)")) -> ()  [unwired: 2 in, 2 out]
          }
          frame #4 {
            n1082 = Wait (ms)(milliseconds to wait=u32 100) -> ()  [unwired: 1 out]
          }
          frame #5 {
            n1083 = property on="Trap Raster Scan" class="Bool (strict)"("Val(Sgnl)"=TRUE ("Value (Signaling)")) -> ()  [unwired: 2 in, 2 out]
          }
          frame #6 {
            n1084 = Wait (ms)(milliseconds to wait=u32 1000) -> ()  [unwired: 1 out]
          }
          frame #7 {
            n1085 = while {
              stop <- w1552 stop-if-true
              n1086 = local read "Raster Scanning..."() -> (w1554:bool)
              n1087 = local read "Saving..."() -> (w1553:bool)
              n1088 = Not(x=w1553) -> (.not. x?=w1550:bool)
              n1089 = Not(x=w1554) -> (.not. x?=w1551:bool)
              n1090 = And(x=w1551, y=w1550) -> (x .and. y?=w1552:bool)
            }
          }
          frame #8 {
            n1091 = property on="Save ave N" class="DigNum (strict)"("Val(Sgnl)"=w1555) -> ()  [unwired: 2 in, 2 out]
          }
        }
      }
      event "Step Size (nm)": Value Change {
        n1092 = event-data() -> ()  [unwired: 1 in, 5 out]
        n1093 = flat-sequence {
          frame #0 {
            n1094 = property on="Saved AOD Raster Scan Parameter Sets" class="Arr (strict)"("Index Values"=u32[] [1]) -> ()  [unwired: 2 in, 2 out]
          }
          frame #1 {
            n1095 = Multiply(x="N Steps", y="Step Size (nm)") -> (x*y=w1557:dbl)
            n1096 = property on="Scan Speed AOD (nm/s) 2" class="DigNum (strict)"("Value"="Step Size (nm)") -> ()  [unwired: 2 in, 2 out]
            n1097 = property on="Step Size AOD (nm) 2" class="DigNum (strict)"("Value"="Step Size (nm)") -> ()  [unwired: 2 in, 2 out]
            n1098 = property on="Scan Range AOD (nm) 2" class="DigNum (strict)"("Value"=w1557) -> ()  [unwired: 2 in, 2 out]
          }
        }
      }
      event "Take Detection Laser\nImage": Value Change {
        n1099 = event-data() -> ()  [unwired: 1 in, 5 out]
        n1100 = flat-sequence {
          tunnel: [w1585] -> w1575
          tunnel: [w1584] -> w1568
          tunnel: [w1583] -> w1560
          tunnel: [w1588] -> w1576
          tunnel: w1575 -> [w1588]
          tunnel: [w1587] -> w1569
          tunnel: w1568 -> [w1587]
          tunnel: [w1586] -> w1561
          tunnel: w1560 -> [w1586]
          tunnel: [w1592] -> w1577
          tunnel: w1576 -> [w1592]
          tunnel: [w1591] -> w1570
          tunnel: w1569 -> [w1591]
          tunnel: [w1590] -> w1562
          tunnel: w1561 -> [w1590]
          tunnel: [w1598] -> w1578
          tunnel: w1577 -> [w1598]
          tunnel: [w1597] -> w1571
          tunnel: w1570 -> [w1597]
          tunnel: [w1596] -> w1563
          tunnel: w1562 -> [w1596]
          tunnel: [w1602] -> w1579
          tunnel: w1578 -> [w1602]
          tunnel: [w1601] -> w1572
          tunnel: w1571 -> [w1601]
          tunnel: [w1600] -> w1564
          tunnel: w1563 -> [w1600]
          tunnel: [w1606] -> w1580
          tunnel: w1579 -> [w1606]
          tunnel: [w1605] -> w1573
          tunnel: w1572 -> [w1605]
          tunnel: [w1604] -> w1565
          tunnel: w1564 -> [w1604]
          tunnel: [w1610] -> w1581
          tunnel: w1580 -> [w1610]
          tunnel: [w1609] -> w1574
          tunnel: w1573 -> [w1609]
          tunnel: [w1608] -> w1566
          tunnel: w1565 -> [w1608]
          tunnel: w1581 -> [w1616]
          tunnel: w1574 -> [w1615]
          tunnel: [w1613] -> w1567
          tunnel: w1566 -> [w1613]
          tunnel: w1567 -> [w1617]
          frame #0 {
            n1101 = local read "Laser interlacing mode"() -> (w1584:enum32{"Laser ON", "Laser OFF", "Interlace"})
            n1102 = local read "Green FB On/Off"() -> (w1583:bool)
            n1103 = local read "Green Laser ON"() -> (w1585:bool)
          }
          frame #1 {
            n1104 = property on="Green FB On/Off" class="Bool (strict)"("Val(Sgnl)"=FALSE ("Value (Signaling)")) -> ()  [unwired: 2 in, 2 out]
          }
          frame #2 {
            n1105 = property on="Green Laser ON" class="Bool (strict)"("Val(Sgnl)"=TRUE ("Value (Signaling)")) -> ()  [unwired: 2 in, 2 out]
            n1106 = property on="Flip Green Filter" class="Bool (strict)"("Val(Sgnl)"=TRUE ("Value (Signaling)")) -> ()  [unwired: 2 in, 2 out]
            n1107 = property on="Laser interlacing mode" class="RadioBtnsControl (strict)"("Val(Sgnl)"=enum32{"Laser ON", "Laser OFF", "Interlace"}."Laser ON" ("Value (Signaling)")) -> ()  [unwired: 2 in, 2 out]